vi "UHR-Fleezers Control (host) - 12.0.vi"() -> ()   [LabVIEW 2014] (continued)
            # "N total cycles"
            # "N steps"
            # "V_int"
            n2516 = local read "Scan Range (nm)"() -> (w4828:dbl)
            n2517 = local read "Number of F/B Scans (AOD)"() -> (w4845:u16)
            n2518 = Sign(1:w4828) -> (0:w4827:dbl)
            n2519 = Compound Arithmetic op=MULTIPLY(w4828, "MCL Step Position Ratio", "MCL/AOM Scale Tweak") -> (w4832:dbl)
            n2520 = Negate(x=w4827) -> (-x=w4824:dbl)
            n2521 = Multiply(x=w4824, y="MCL Step Increment (V_int)") -> (x*y=w4826:dbl)
            n2522 = Divide(x=w4832, y="MCL X Cal (nm/V)") -> (x/y=w4838:dbl)
            n2523 = Multiply(x=32767.0 ("y"), y=w4838) -> (x*y=w4844:dbl)
            n2524 = local read "Total Counts (ticks)"() -> (w4829:u32)
            n2525 = local read "Cycles/step (AOD)"() -> (w4840:u64)
            n2526 = local read "Scan steps (AOD)"() -> (w4841:u64)
            n2527 = Divide(x=w4844, y=10.0) -> (x/y=w4837:dbl)
            n2528 = Divide(x=w4837, y="MCL Step Increment (V_int)") -> (x/y=w4835:dbl)
            n2529 = Absolute Value(x=w4835) -> (abs(x)=w4823:dbl)
            n2530 = Compound Arithmetic op=MULTIPLY(w4841, w4840, w4829) -> (w4836:u64)
            n2531 = local write "wait to reset values"(w4851) -> ()
            n2532 = local write "MCL Scanning"(w4851) -> ()
            n2533 = Divide(x=w4836, y=w4823) -> (x/y=w4833:dbl)
            "MCL Count" <- w4833
            n2534 = xnode "Read/Write Control"("FPGA VI Reference In"=w4850, "error in"=w4849, "Scan steps (MCL)"=w4823, "Number of scans (MCL)"=w4845, "Cycles per step (MCL)"=u64 1, "Scan freq.  increment (MCL)"=w4826, "1D or 2D Scan?"=w4846, "MCL Scan Axis"=w4846, "Cont. Scan (MCL)"=w4846, "MCL count"=w4833) -> ("FPGA VI Reference Out"=w4848:T22, "error out"=w4847:errorcluster)
            n2535 = xnode "Read/Write Control"("FPGA VI Reference In"=w4848, "error in"=w4847, "AI to FIFO"=w4851, "APD to FIFO"=w4851, "Start scan"=w4851, "Start scan (MCL)"=w4851) -> ("FPGA VI Reference Out"=w4853:T22, "error out"=w4852:errorcluster)
          }
        }
        "Raster Scanning..." <- TRUE ("Scanning...")
      }
    }
    n2536 = local read "Flushing P3"() -> (w3628:bool)
    n2537 = case "Keep track of when Harvard Pump 3 is done flushing" shown="True" w3628 {
      frame False {
      }
      frame True {
        n2538 = local read "Flush rate (uL/m) P3"() -> (w4011:dbl)
        n2539 = local read "DMA Update Period (s)"() -> (w4005:dbl)
        n2540 = local read "HP3 Flush Time (s)"() -> (w4019:dbl)
        n2541 = Divide(x=w4011, y=60.0) -> (x/y=w4006:dbl)
        n2542 = feedback #6(0) -> (w4017:i32)
        n2543 = Increment(x=w4017) -> (x+1=w4012:i32)
        n2544 = Divide(x=w4019, y=w4005) -> (x/y=w4013:dbl)
        n2545 = Multiply(x=w4005, y=w4006) -> (x*y=w4004:dbl)
        n2546 = Greater?(x=w4012, y=w4013) -> (0:w4016:bool)
        n2547 = feedback #7(0.0) -> (w4007:dbl)
        n2548 = Compound Arithmetic op=MULTIPLY(w4005, w4012, w4006) -> (→"P3 Flush Volume (uL)":dbl)
        n2549 = case shown="True" w4016 {
          tunnel: w4012 -> [w4020 _]
          tunnel: [w4020 0] -> w4015
          frame False {
          }
          frame True {
            w4021 = FALSE ("Flushing P3")
            n2550 = local write "Inject Pump 3"(w4021) -> ()
            n2551 = local write "Flushing P3"(w4021) -> ()
            n2552 = property on="Clear Volume P3" class="Bool (strict)"("Val(Sgnl)"=TRUE ("Value (Signaling)")) -> ()  [unwired: 2 in, 2 out]
          }
        }
        n2553 = feedback-in #6(w4015) -> ()
        n2554 = Divide(x=w4012, y=w4013) -> (x/y=→"P3 Flushing Bar":dbl)
        n2555 = Add(x=w4004, y=w4007) -> (x+y=w4008:dbl)
        "Total Volume\nFlowed P3 (uL)" <- w4008
        n2556 = feedback-in #7(w4008) -> ()
      }
    }
    n2557 = And(x="Save scans", y=w3846) -> (x .and. y?=w3885:bool)
    n2558 = local read "Flushing samp"() -> (w3621:bool)
    n2559 = case shown="True" w3621 {
      frame False {
      }
      frame True {
        n2560 = local read "DMA Update Period (s)"() -> (w3964:dbl)
        n2561 = local read "Flush rate (mL/m)"() -> (w3976:dbl)
        n2562 = local read "Samp Flush Time (s)"() -> (w3977:dbl)
        n2563 = Divide(x=w3976, y=60.0) -> (x/y=w3963:dbl)
        n2564 = feedback #8(0) -> (w3969:i32)
        n2565 = Increment(x=w3969) -> (x+1=w3968:i32)
        n2566 = Divide(x=w3977, y=w3964) -> (x/y=w3973:dbl)
        n2567 = Multiply(x=w3964, y=w3963) -> (x*y=w3962:dbl)
        n2568 = Greater?(x=w3968, y=w3973) -> (0:w3972:bool)
        n2569 = feedback #9(0.0) -> (w3965:dbl)
        n2570 = Compound Arithmetic op=MULTIPLY(w3964, w3968, w3963) -> (→"Samp Volume (uL)":dbl)
        n2571 = Divide(x=w3968, y=w3973) -> (x/y=→"Samp flush bar":dbl)
        n2572 = case shown="True" w3972 {
          tunnel: [w3978 0] -> w3971
          tunnel: w3968 -> [w3978 _]
          frame False {
          }
          frame True {
            w3981 = FALSE ("Flushing samp")
            n2573 = local write "Sample Channel\nFlow"(w3981) -> ()
            n2574 = local write "Flushing samp"(w3981) -> ()
            n2575 = property on="Clear Volume" class="Bool (strict)"("Val(Sgnl)"=TRUE) -> ()  [unwired: 2 in, 2 out]
          }
        }
        n2576 = feedback-in #8(w3971) -> ()
        n2577 = Add(x=w3962, y=w3965) -> (x+y=w3966:dbl)
        "Total Volume\nFlowed Samp (uL)" <- w3966
        n2578 = feedback-in #9(w3966) -> ()
      }
    }
    n2579 = Compound Arithmetic op=OR("Start MCL Scan", "Confocal\nImage", "Confocal\nLinescan") -> (w3844:bool)
    n2580 = And(x="Save Data (MCL)", y=w3844) -> (x .and. y?=w3884:bool)
    n2581 = case "Start MCL raster scan" shown="True" w3844 {
      tunnel: w3612 -> [w4426 w4442]
      tunnel: w3886 -> [w4425 w4441]
      tunnel: [w4426 w4437] -> w3619
      tunnel: [w4425 w4436] -> w3617
      tunnel: [FALSE w4435] -> w3870
      tunnel: "Start MCL Scan" -> [_ w4430]
      tunnel: "Confocal\nImage" -> [_ w4429]
      tunnel: "Confocal\nLinescan" -> [_ _]
      frame False {
      }
      frame True {
        w4435 = TRUE
        n2582 = case shown="True" "Restart DMA? (MCL)" {
          tunnel: [w4487 w4489] -> w4440
          tunnel: [w4486 w4488] -> w4439
          tunnel: w4442 -> [w4487 w4492]
          tunnel: w4441 -> [w4486 w4491]
          frame False {
          }
          frame True {
            n2583 = call "reset FPGA DMA.vi"("error in"=w4491, "FPGA VI Reference In"=w4492) -> ("error out"=w4488:errorcluster, "FPGA VI Reference Out"=w4489:T22)
            n2584 = local write "Overflow (data lost)"(FALSE ("Overflow (data lost)")) -> ()
          }
        }
        n2585 = case shown="False" w4430 {
          selector: w4430 -> [_ w4446]
          tunnel: w4429 -> [w4445 _]
          tunnel: [w4445 w4446] -> w4428
          frame False {
            n2586 = property on="2D or 1D Scan" class="Bool (strict)"("Val(Sgnl)"=w4445) -> ()  [unwired: 2 in, 2 out]
            n2587 = property on="Confocal\nImage" class="Bool (strict)"("Value"=FALSE ("Start Confocal Map")) -> ()  [unwired: 2 in, 2 out]
          }
          frame True {
          }
        }
        n2588 = local write "MCL Scanning"(w4435) -> ()
        n2589 = local read "AO1"() -> (w4432:dbl)
        n2590 = local read "AO2"() -> (w4431:dbl)
        n2591 = case shown="True" "Center Scan" {
          tunnel: w4440 -> [w4453 w4485]
          tunnel: w4439 -> [w4452 w4484]
          tunnel: [w4451 w4483] -> w4437
          tunnel: [w4450 w4482] -> w4436
          tunnel: [w4448 w4469] -> w4434
          tunnel: [w4447 w4468] -> w4433
          tunnel: w4432 -> [w4448 w4474]
          tunnel: w4431 -> [w4447 w4477]
          tunnel: w4428 -> [_ _]
          frame False {
            w4449 = TRUE ("AI to FIFO")
            n2592 = xnode "Read/Write Control"("FPGA VI Reference In"=w4453, "error in"=w4452, "AI to FIFO"=w4449, "APD to FIFO"=w4449, "Start scan (MCL)"=w4449) -> ("FPGA VI Reference Out"=w4451:T22, "error out"=w4450:errorcluster)
          }
          frame True {
            w4481 = TRUE ("AI to FIFO")
            n2593 = local read "Scan steps (MCL)"() -> (w4460:u64)
            n2594 = local read "Scan lines (y)"() -> (w4456:u64)
            n2595 = local read "Fast Scan Dir"() -> (w4467:bool)
            n2596 = local read "Actual MCL Inc (V)"() -> (w4457:dbl)
            n2597 = Decrement(x=w4456) -> (x-1=w4455:u64)
            n2598 = Decrement(x=w4460) -> (x-1=w4459:u64)
            n2599 = Multiply(x=w4457, y=w4455) -> (x*y=w4454:dbl)
            n2600 = Divide(x=w4454, y=2.0) -> (x/y=w4464:dbl)
            n2601 = Multiply(x=w4457, y=w4459) -> (x*y=w4458:dbl)
            n2602 = Divide(x=w4458, y=2.0) -> (x/y=w4463:dbl)
            n2603 = Select(t=w4463, s=w4467, f=w4464) -> (s? t:f=w4462:dbl)
            n2604 = Select(t=w4464, s=w4467, f=w4463) -> (s? t:f=w4466:dbl)
            n2605 = Subtract(x=w4474, y=w4466) -> (x-y=w4465:dbl)
            n2606 = Subtract(x=w4477, y=w4462) -> (x-y=w4461:dbl)
            n2607 = local read "2D or 1D Scan"() -> (w4479:bool)
            n2608 = Not(x=w4467) -> (.not. x?=w4473:bool)
            n2609 = Not(x=w4479) -> (.not. x?=w4475:bool)
            n2610 = And(x=w4467, y=w4475) -> (x .and. y?=w4476:bool)
            n2611 = And(x=w4475, y=w4473) -> (x .and. y?=w4478:bool)
            n2612 = Select(t=w4477, s=w4478, f=w4461) -> (s? t:f=w4468:dbl)
            n2613 = Select(t=w4474, s=w4476, f=w4465) -> (s? t:f=w4469:dbl)
            n2614 = call "Volt to I16.vi"("Voltage In"=w4469) -> ("I16 Voltage Out"=w4472:i16)
            n2615 = call "Volt to I16.vi"("Voltage In"=w4468) -> ("I16 Voltage Out"=w4471:i16)
            n2616 = xnode "Read/Write Control"("FPGA VI Reference In"=w4485, "error in"=w4484, "AI to FIFO"=w4481, "APD to FIFO"=w4481, "Start scan (MCL)"=w4481, "AO1"=w4472, "AO2"=w4471) -> ("FPGA VI Reference Out"=w4483:T22, "error out"=w4482:errorcluster)
          }
        }
        "Initial Y" <- w4434
        "Initial X" <- w4433
        n2617 = local write "Tab Control 6"(T3."Imaging" ("Tab Control 6")) -> ()
        "wait to reset values" <- w4435
      }
    }
    n2618 = case shown="True" "Wiggle" {
      selector: "Wiggle" -> [w3935 _]
      tunnel: w3619 -> [w3937 w3950]
      tunnel: [w3934 w3953] -> w3618
      tunnel: w3617 -> [w3936 w3948]
      tunnel: [w3933 w3952] -> w3616
      frame False {
        n2619 = xnode "Read/Write Control"("FPGA VI Reference In"=w3937, "error in"=w3936, "Wiggle trap 1"=w3935) -> ("FPGA VI Reference Out"=w3934:T22, "error out"=w3933:errorcluster)
      }
      frame True {
        w3942 = FALSE ("Abort wiggle")
        w3946 = TRUE
        n2620 = local read "Restart DMA? (AOD)"() -> (w3951:bool)
        n2621 = case shown="True" w3951 {
          tunnel: w3950 -> [w3955 w3960]
          tunnel: [w3955 w3959] -> w3949
          tunnel: w3948 -> [w3954 w3958]
          tunnel: [w3954 w3957] -> w3947
          frame False {
          }
          frame True {
            n2622 = local write "Overflow (data lost)"(FALSE) -> ()
            n2623 = call "reset FPGA DMA.vi"("error in"=w3958, "FPGA VI Reference In"=w3960) -> ("error out"=w3957:errorcluster, "FPGA VI Reference Out"=w3959:T22)
          }
        }
        n2624 = local write "Wiggle"(FALSE) -> ()
        n2625 = xnode "Read/Write Control"("FPGA VI Reference In"=w3949, "error in"=w3947, "AI to FIFO"=w3946, "APD to FIFO"=w3946, "Wiggle trap 1"="Wiggle T1", "Wiggle freq 1 (Hz)"="Wiggle freq 1 (Hz)", "Wiggle amp 1"="Wiggle amp 1 (units?)", "Abort wiggle 1"=w3942, "Wiggle trap 2"="Wiggle T2", "Abort wiggle 2"=w3942, "Wiggle freq 2 (Hz)"="Wig Freq 2 (Hz)", "Wiggle amp 2"="Wig amp 2") -> ("FPGA VI Reference Out"=w3953:T22, "error out"=w3952:errorcluster)
      }
    }
    n2626 = local read "Trap Pos Elements/DMA read"() -> (w3602:u32)
    n2627 = local read "Trap AI Elements/DMA read"() -> (w3596:u32)
    n2628 = local read "APD Elements/DMA read"() -> (w3604:u32)
    n2629 = xnode "Get APD Data"("FPGA VI Reference In"=w3618, "error in"=w3616, "Number of Elements"=w3604, "Timeout (ms)"=-1) -> ("Data"=w3780:u32[], "Elements Remaining"=→"APD FIFO Elements Remaining":u32)  [unwired: 2 out]
    n2630 = xnode "Invoke Method"("FPGA VI Reference In"=w3618, "error in"=w3616, "Number of Elements"=w3602, "Timeout (ms)"=-1) -> ("Data"=w3711:u16[], "Elements Remaining"=→"Trap Pos FIFO El Remaining":u32)  [unwired: 2 out]
    n2631 = xnode "Get Trap Data"("FPGA VI Reference In"=w3618, "error in"=w3616, "Number of Elements"=w3596, "Timeout (ms)"=-1 ("Timeout")) -> ("FPGA VI Reference Out"=w3649:T22, "error out"=w3648:errorcluster, "Data"=w3712:i16[], "Elements Remaining"=w3595:u32)
    "FIFO El. Rem." <- w3595
    n2632 = local read "Trap AI FIFO Depth"() -> (w3930:u32)
    n2633 = Subtract(x=w3930, y=w3596) -> (x-y=w3929:u32)
    n2634 = Decimate 1D Array(w3711) -> (w3600:u16[], w3598:u16[], w3599:u16[])
    n2635 = Divide(x=w3595, y=w3929) -> (x/y=w3928:dbl)
    "Buffer Status" <- w3928
    n2636 = To Unsigned Long Integer(number=w3600) -> (unsigned 32bit integer=w3710:u32[])
    n2637 = Join Numbers(hi=w3598, lo=w3599) -> ((hi.lo)=w3709:u32[])
    n2638 = Equal?(x=w3928, y=1.0) -> (x = y?=w3926:bool)
    n2639 = Join Numbers(hi=w3710, lo=w3709) -> ((hi.lo)=w3703:u64[])
    n2640 = call "IR AOM word to freq - vec.vi"("Frequency Word In (double vec)"=w3703) -> ("Frequency Out"=w3746:dbl[])
    n2641 = case "Alert buffer overflow" shown="True" w3926 {
      frame False {
      }
      frame True {
        n2642 = call <vilib>:"Beep.vi"() -> ()  [unwired: 3 in, 9 out]
        "Overflow (data lost)" <- TRUE ("Overflow (data lost)")
      }
    }
    n2643 = Decimate 1D Array(w3746) -> (w3745:dbl[], w3744:dbl[])
    n2644 = Build Array(w3745, w3744) -> (w3743:dbl[][])
    n2645 = local read "Trap Sets"() -> (w3810:u32)
    n2646 = case "Deinterlace trap data, average down PSD" shown="2" w3810 {
      tunnel: w3712 -> [w4518 w4587]
      tunnel: [w4521 w4584] -> w3803
      tunnel: [w4518 w4586] -> w3706
      tunnel: "Detector Type" -> [w4523 w4582]
      tunnel: [w4522 w4585] -> w3802
      tunnel: [w4520 w4583] -> w3903
      frame 1, Default {
        n2647 = Divide(x=w4518, y=3276.7) -> (x/y=w4519:dbl[])
        n2648 = Decimate 1D Array(w4519) -> (w4532:dbl[], w4531:dbl[], w4530:dbl[], w4529:dbl[], w4528:dbl[], w4527:dbl[], w4526:dbl[], w4525:dbl[])
        n2649 = case shown="\"IR-QPD + PSD + FB-QPD position\"" w4523 {
          tunnel: w4532 -> [w4556 w4581]
          tunnel: w4531 -> [w4555 w4580]
          tunnel: w4530 -> [w4540 w4558]
          tunnel: w4529 -> [w4541 w4568]
          tunnel: w4528 -> [w4554 w4579]
          tunnel: w4527 -> [w4553 w4578]
          tunnel: w4526 -> [w4537 w4559]
          tunnel: w4525 -> [w4536 w4557]
          tunnel: [w4535 w4565] -> w4522
          tunnel: [w4534 w4564] -> w4521
          tunnel: [w4533 w4563] -> w4520
          frame "IR-QPD + PSD + FB-QPD", Default {
            w4533 = 0  # Channel pattern
            n2650 = Divide(x=w4556, y=w4541) -> (x/y=w4543:dbl[])
            n2651 = Divide(x=w4555, y=w4541) -> (x/y=w4542:dbl[])
            n2652 = Divide(x=w4554, y=w4537) -> (x/y=w4539:dbl[])
            n2653 = Divide(x=w4553, y=w4536) -> (x/y=w4538:dbl[])
            n2654 = Build Array(w4543, w4542, w4541, w4540, w4539, w4538, w4537, w4536) -> (w4534:dbl[][])
            n2655 = Bundle("T1 Y", "T1 X", "T1 Sum", "FB Sum", "PSD Y", "PSD X", "PSD Y Sum", "PSD X Sum") -> (w4552:T47)  [unwired: 1 out]
            n2656 = Cluster To Array(cluster=w4552) -> (array=w4535:string[])
          }
          frame "IR-QPD + PSD + FB-QPD position" {
            w4563 = 3  # Channel pattern
            n2657 = Negate(x=w4559) -> (-x=w4560:dbl[])
            n2658 = Divide(x=w4581, y=w4568) -> (x/y=w4570:dbl[])
            n2659 = Divide(x=w4580, y=w4568) -> (x/y=w4569:dbl[])
            n2660 = Divide(x=w4579, y=w4559) -> (x/y=w4567:dbl[])
            n2661 = Divide(x=w4578, y=w4560) -> (x/y=w4566:dbl[])
            n2662 = Build Array(w4570, w4569, w4568, w4557, w4558, w4567, w4566, w4559) -> (w4564:dbl[][])
            n2663 = Bundle("T1 Y", "T1 X", "T1 Sum", "FB X", "FB Sum", "PSD Y", "PSD X", "PSD Y Sum") -> (w4577:T47)  [unwired: 1 out]
            n2664 = Cluster To Array(cluster=w4577) -> (array=w4565:string[])
          }
        }
      }
      frame 2 {
        n2665 = case shown="\"IR-QPD + PSD + FB-QPD XY positions\"" w4582 {
          tunnel: w4587 -> [w4649 w4716 w4785]
          tunnel: [w4600 w4712 w4730] -> w4586
          tunnel: [w4625 w4704 w4771] -> w4585
          tunnel: [w4624 w4671 w4742] -> w4584
          tunnel: [w4620 w4702 w4769] -> w4583
          frame "IR-QPD + PSD + FB-QPD", Default {
            w4620 = 1  # Channel pattern
            # "time average x2 the 4th signal and the 4 psd signals (detection laser)"
            # "deinterlace 3 signals from qpd"
            n2666 = Decimate 1D Array(w4649) -> (w4648:i16[], w4647:i16[], w4623:i16[], w4646:i16[], w4599:i16[], w4598:i16[], w4597:i16[], w4596:i16[])
            n2667 = Decimate 1D Array(w4623) -> (w4589:i16[], w4588:i16[])
            n2668 = Decimate 1D Array(w4648) -> (w4595:i16[], w4594:i16[])
            n2669 = Decimate 1D Array(w4647) -> (w4593:i16[], w4591:i16[])
            n2670 = Decimate 1D Array(w4646) -> (w4592:i16[], w4590:i16[])
            n2671 = call "downsample 1D array - double.vi"("Ave N"=2.0, "Array In"=w4599) -> ("Array Out"=w4641:dbl[])  [unwired: 1 out]
            n2672 = call "downsample 1D array - double.vi"("Ave N"=2.0, "Array In"=w4598) -> ("Array Out"=w4626:dbl[])  [unwired: 1 out]
            n2673 = call "downsample 1D array - double.vi"("Ave N"=2.0, "Array In"=w4597) -> ("Array Out"=w4640:dbl[])  [unwired: 1 out]
            n2674 = call "downsample 1D array - double.vi"("Ave N"=2.0, "Array In"=w4596) -> ("Array Out"=w4639:dbl[])  [unwired: 1 out]
            n2675 = Interleave 1D Arrays(w4595, w4593, w4592, w4594, w4591, w4590, w4589, w4588, w4641, w4626, w4640, w4639) -> (w4638:dbl[])
            n2676 = Divide(x=w4638, y=3276.7) -> (x/y=w4637:dbl[])
            n2677 = Decimate 1D Array(w4637) -> (w4636:dbl[], w4635:dbl[], w4634:dbl[], w4633:dbl[], w4632:dbl[], w4631:dbl[], w4622:dbl[], w4621:dbl[], w4630:dbl[], w4629:dbl[], w4628:dbl[], w4627:dbl[])
            n2678 = Divide(x=w4636, y=w4634) -> (x/y=w4607:dbl[])
            n2679 = Divide(x=w4635, y=w4634) -> (x/y=w4606:dbl[])
            n2680 = Divide(x=w4633, y=w4631) -> (x/y=w4605:dbl[])
            n2681 = Divide(x=w4632, y=w4631) -> (x/y=w4604:dbl[])
            n2682 = Divide(x=w4630, y=w4628) -> (x/y=w4603:dbl[])
            n2683 = Divide(x=w4629, y=w4627) -> (x/y=w4602:dbl[])
            n2684 = Build Array(w4607, w4606, w4634, w4605, w4604, w4631, w4622, w4621, w4603, w4602, w4628, w4627) -> (w4624:dbl[][])
            n2685 = Bundle("T1 Y", "T1 X", "T1 Sum", "T2 Y", "T2 X", "T2 Sum", "T1 FB Sum", "T2 FB Sum", "PSD Y", "PSD X", "PSD Y Sum", "PSD X Sum") -> (w4608:T48)  [unwired: 1 out]
            n2686 = To Word Integer(number=w4638) -> (16bit integer=w4600:i16[])
            n2687 = Cluster To Array(cluster=w4608) -> (array=w4625:string[])
          }
          frame "IR-QPD + PSD + FB-QPD X position" {
            w4702 = 2  # Channel pattern
            # "time average x2 the 3 psd signals (detection laser)"
            # "deinterlace 3 signals from qpds"
            n2688 = Decimate 1D Array(w4716) -> (w4715:i16[], w4714:i16[], w4703:i16[], w4713:i16[], w4663:i16[], w4662:i16[], w4661:i16[], w4690:i16[])
            n2689 = Decimate 1D Array(w4703) -> (w4653:i16[], w4651:i16[])
            n2690 = Decimate 1D Array(w4715) -> (w4660:i16[], w4657:i16[])
            n2691 = Decimate 1D Array(w4714) -> (w4659:i16[], w4656:i16[])
            n2692 = Decimate 1D Array(w4713) -> (w4658:i16[], w4655:i16[])
            n2693 = Decimate 1D Array(w4690) -> (w4654:i16[], w4652:i16[])
            n2694 = call "downsample 1D array - I16.vi"("Ave N"=2.0, "Array In"=w4663) -> ("Array Out"=w4668:i16[])  [unwired: 1 in]
            n2695 = call "downsample 1D array - I16.vi"("Ave N"=2.0, "Array In"=w4661) -> ("Array Out"=w4664:i16[])  [unwired: 1 in]
            n2696 = call "downsample 1D array - I16.vi"("Ave N"=2.0, "Array In"=w4662) -> ("Array Out"=w4666:i16[])  [unwired: 1 in]
            n2697 = Interleave 1D Arrays(w4660, w4659, w4658, w4657, w4656, w4655, w4654, w4653, w4652, w4651, w4668, w4666, w4664) -> (w4712:i16[])
            n2698 = Divide(x=w4712, y=3276.7) -> (x/y=w4711:dbl[])
            n2699 = Decimate 1D Array(w4711) -> (w4710:dbl[], w4709:dbl[], w4708:dbl[], w4707:dbl[], w4706:dbl[], w4705:dbl[], w4682:dbl[], w4680:dbl[], w4679:dbl[], w4677:dbl[], w4676:dbl[], w4675:dbl[], w4672:dbl[])
            n2700 = Negate(x=w4672) -> (-x=w4670:dbl[])
            n2701 = Divide(x=w4676, y=w4672) -> (x/y=w4674:dbl[])
            n2702 = Divide(x=w4675, y=w4670) -> (x/y=w4673:dbl[])
            n2703 = Divide(x=w4710, y=w4708) -> (x/y=w4694:dbl[])
            n2704 = Divide(x=w4709, y=w4708) -> (x/y=w4693:dbl[])
            n2705 = Divide(x=w4707, y=w4705) -> (x/y=w4692:dbl[])
            n2706 = Divide(x=w4706, y=w4705) -> (x/y=w4691:dbl[])
            n2707 = Divide(x=w4682, y=w4680) -> (x/y=w4681:dbl[])
            n2708 = Divide(x=w4679, y=w4677) -> (x/y=w4678:dbl[])
            n2709 = Build Array(w4694, w4693, w4708, w4692, w4691, w4705, w4681, w4680, w4678, w4677, w4674, w4673, w4672) -> (w4671:dbl[][])
            n2710 = Bundle("T1 Y", "T1 X", "T1 Sum", "T2 Y", "T2 X", "T2 Sum", "T1 FB X", "T1 FB Sum", "T2 FB X", "T2 FB Sum", "PSD Y", "PSD X", "PSD Y Sum") -> (w4695:T49)  [unwired: 1 out]
            n2711 = Cluster To Array(cluster=w4695) -> (array=w4704:string[])
          }
          frame "IR-QPD + PSD + FB-QPD XY positions" {
            w4769 = 4  # Channel pattern
            # "time average x2 the 3 psd signals (detection laser)"
            # "deinterlace 3 signals from qpds"
            n2712 = Decimate 1D Array(w4785) -> (w4784:i16[], w4783:i16[], w4770:i16[], w4782:i16[], w4740:i16[], w4758:i16[])  [unwired: 2 out]
            n2713 = Decimate 1D Array "Feedback Sum"(w4770) -> (w4721:i16[], w4718:i16[])
            n2714 = Decimate 1D Array "QPD Y"(w4784) -> (w4729:i16[], w4726:i16[])
            n2715 = Decimate 1D Array "QPD X"(w4783) -> (w4728:i16[], w4725:i16[])
            n2716 = Decimate 1D Array "Feedback Y"(w4740) -> (w4723:i16[], w4720:i16[])
            n2717 = Decimate 1D Array "QPD Sum"(w4782) -> (w4727:i16[], w4724:i16[])
            n2718 = Decimate 1D Array "Feedback X"(w4758) -> (w4722:i16[], w4719:i16[])
            n2719 = call "downsample 1D array - double.vi"("Ave N"=2.0) -> ("Array Out"=w4757:dbl[])  [unwired: 1 in, 1 out]
            n2720 = call "downsample 1D array - double.vi"("Ave N"=2.0) -> ("Array Out"=w4756:dbl[])  [unwired: 1 in, 1 out]
            n2721 = Interleave 1D Arrays(w4729, w4728, w4727, w4726, w4725, w4724, w4723, w4722, w4721, w4720, w4719, w4718, w4757, w4756) -> (w4779:dbl[])
            n2722 = Divide(x=w4779, y=3276.7) -> (x/y=w4778:dbl[])
            n2723 = Decimate 1D Array(w4778) -> (w4777:dbl[], w4776:dbl[], w4775:dbl[], w4774:dbl[], w4773:dbl[], w4772:dbl[], w4737:dbl[], w4749:dbl[], w4735:dbl[], w4736:dbl[], w4747:dbl[], w4733:dbl[], w4745:dbl[], w4743:dbl[])
            n2724 = Negate(x=w4743) -> (-x=w4741:dbl[])
            n2725 = Divide(x=w4745, y=w4741) -> (x/y=w4744:dbl[])
            n2726 = Divide(x=w4736, y=w4733) -> (x/y=w4732:dbl[])
            n2727 = Divide(x=w4737, y=w4735) -> (x/y=w4734:dbl[])
            n2728 = Divide(x=w4777, y=w4775) -> (x/y=w4762:dbl[])
            n2729 = Divide(x=w4776, y=w4775) -> (x/y=w4761:dbl[])
            n2730 = Divide(x=w4774, y=w4772) -> (x/y=w4760:dbl[])
            n2731 = Divide(x=w4773, y=w4772) -> (x/y=w4759:dbl[])
            n2732 = Divide(x=w4749, y=w4735) -> (x/y=w4748:dbl[])
            n2733 = Divide(x=w4747, y=w4733) -> (x/y=w4746:dbl[])
            n2734 = Build Array(w4762, w4761, w4775, w4760, w4759, w4772, w4734, w4748, w4735, w4732, w4746, w4733, w4744, w4743) -> (w4742:dbl[][])
            n2735 = Bundle("T1 Y", "T1 X", "T1 Sum", "T2 Y", "T2 X", "T2 Sum", "T1 FB Y", "T1 FB X", "T1 FB Sum", "T2 FB Y", "T2 FB X", "T2 FB Sum", "PSD X", "PSD Y Sum") -> (w4731:T50)  [unwired: 1 out]
            n2736 = To Word Integer(number=w4779) -> (16bit integer=w4730:i16[])
            n2737 = Cluster To Array(cluster=w4731) -> (array=w4771:string[])
          }
        }
      }
    }
    "AI labels" <- w3802
    n2738 = Decimate 1D Array(w3780) -> (w3590:u32[], w3591:u32[])
    n2739 = local read "DMA Update Period (s)"() -> (w3811:dbl)
    n2740 = Build Array(w3590, w3591) -> (w3594:u32[][])
    n2741 = local read "Data Period (s)"() -> (w3665:dbl)
    n2742 = local read "BD 1 Frequency 2 (MHz)"() -> (w3698:dbl)
    n2743 = local read "BD 1 Frequency 1 (MHz)"() -> (w3699:dbl)
    n2744 = Decimate 1D Array(w3706) -> (w3726:i16[], w3725:i16[], w3723:i16[], w3722:i16[])  [unwired: 9 out]
    n2745 = To Double Precision Float(number=w3594) -> (double precision float=w3868:dbl[][])
    n2746 = local read "APD Integration Time (s)"() -> (w3762:dbl)
    n2747 = Multiply(x=w3665, y="Trap Pos. Disp. Downsample") -> (x*y=w3663:dbl)
    n2748 = Divide(x=w3726, y=w3725) -> (x/y=w3727:dbl[])
    n2749 = Divide(x=w3723, y=w3722) -> (x/y=w3724:dbl[])
    n2750 = feedback #10(0.0) -> (w3740:dbl)
    n2751 = Add(x=w3811, y=w3740) -> (x+y=w3905:dbl)
    n2752 = feedback-in #10(w3905) -> ()
    n2753 = local read "AOM X Cal (nm/MHz)"() -> (w3696:dbl)
    n2754 = To Time Stamp(1:w3740) -> (0:w3739:timestamp)
    n2755 = Split 1D Array(array=w3727, index="N El. to Ave.") -> (second subarray=w3730:dbl[])  [unwired: 1 out]
    n2756 = Split 1D Array(array=w3724, index="N El. to Ave.") -> (second subarray=w3729:dbl[])  [unwired: 1 out]
    n2757 = Multiply(x=w3665, y="Trap Disp. Downsample") -> (x*y=w3741:dbl)
    "Display Period (s)" <- w3741
    n2758 = for "Trap AI" {
      tunnel: [w4517] -> w3899 mode=indexing
      tunnel: w3739 -> [w4507]
      tunnel: "Trap Disp. Downsample" -> [w4515]
      tunnel: w3803 -> [w4513] mode=indexing
      tunnel: w3665 -> [w4512]
      tunnel: w3802 -> [w4511] mode=indexing
      tunnel: w3738 -> [w4510]
      tunnel: [w4509] -> w3772 mode=indexing
      tunnel: w3741 -> [w4508]
      workers-P: _ -> [_]
      n2759 = Bundle By Name("Y"=w4513, "dt"=w4512) -> (w4514:waveform(dbl))  [unwired: 1 out]
      n2760 = Set Waveform Attribute(5:w4511, 6:w4510, 7:w4514) -> (3:w4509:waveform(dbl))  [unwired: 1 in, 2 out]
      n2761 = call "downsample 1D array - double.vi"("Ave N"=w4515, "Array In"=w4513) -> ("Array Out"=w4516:dbl[])  [unwired: 1 out]
      n2762 = Bundle By Name(cluster=w4509, "t0"=w4507, "Y"=w4516, "dt"=w4508) -> (w4517:waveform(dbl))
    }
    n2763 = Bundle("BD 1 Frequency 1 (MHz)"=w3699, "BD 1 Frequency 2 (MHz)"=w3698) -> (w3700:T51)  [unwired: 1 out]
    n2764 = call-poly <vilib>:"Mean.vi"("X"=w3729) -> ("mean"=w3717:dbl)  [unwired: 1 out]
    n2765 = call-poly <vilib>:"Mean.vi"("X"=w3730) -> ("mean"=w3718:dbl)  [unwired: 1 out]
    n2766 = Reciprocal(x=w3741) -> (1/x=→"Trap Disp. Freq. (Hz)":dbl)
    n2767 = Cluster To Array(cluster=w3700) -> (array=w3697:dbl[])
    n2768 = local read "Trap X AI1 (DMA)"() -> (w3728:T13)
    n2769 = local read "Data points/scans (MCL)"() -> (w3879:dbl)
    n2770 = To Fixed-Point(number=w3717) -> (fixed-point=w3715:fxp<+/-,16,1>)  [unwired: 1 in]
    n2771 = To Fixed-Point(number=w3718) -> (fixed-point=w3716:fxp<+/-,16,1>)  [unwired: 1 in]
    n2772 = Bundle("Trap 1 Pos.", "Trap 2 Pos.") -> (w3737:cluster{string, string})  [unwired: 1 out]
    n2773 = Bundle By Name(cluster=w3728, "Set 1"=w3716, "Set 2"=w3715) -> (→"Trap X AI1 (DMA)":T13)
    n2774 = Cluster To Array(cluster=w3737) -> (array=w3734:string[])
    n2775 = Bundle("APD 1", "APD 2") -> (w3898:cluster{string, string})  [unwired: 1 out]
    n2776 = Select(t=-1.0, s="Negate Y Axis", f=1.0) -> (s? t:f=w3682:dbl)
    n2777 = for "Trap Position" {
      tunnel: w3743 -> [w4149] mode=indexing
      tunnel: "Trap Pos. Disp. Downsample" -> [w4148]
      tunnel: w3663 -> [w4146]
      tunnel: w3739 -> [w4145]
      tunnel: w3738 -> [w4143]
      tunnel: w3734 -> [w4142] mode=indexing
      tunnel: [w4141] -> w3652 mode=indexing
      tunnel: w3697 -> [w4139] mode=indexing
      tunnel: w3696 -> [w4137]
      tunnel: w3682 -> [w4136]
      n2778 = call "downsample 1D array - double.vi"("Ave N"=w4148, "Array In"=w4149) -> ("Array Out"=w4147:dbl[])  [unwired: 1 out]
      n2779 = Subtract(x=w4147, y=w4139) -> (x-y=w4140:dbl[])
      n2780 = Multiply(x=w4137, y=w4140) -> (x*y=w4138:dbl[])
      n2781 = Multiply(x=w4136, y=w4138) -> (x*y=w4135:dbl[])
      n2782 = Bundle By Name("Y"=w4135, "dt"=w4146, "t0"=w4145) -> (w4144:waveform(dbl))  [unwired: 1 out]
      n2783 = Set Waveform Attribute(5:w4142, 6:w4143, 7:w4144) -> (3:w4141:waveform(dbl))  [unwired: 1 in, 2 out]
    }
    n2784 = Cluster To Array(cluster=w3898) -> (array=w3895:string[])
    n2785 = for "APD" {
      tunnel: w3868 -> [w4493] mode=indexing
      tunnel: w3762 -> [w4504]
      tunnel: [w4500] -> w3768 mode=indexing
      tunnel: "APD Disp. Scale" -> [w4501]
      tunnel: w3738 -> [w4499]
      tunnel: w3895 -> [w4498] mode=indexing
      tunnel: "APD Disp. Downsample" -> [w4495]
      tunnel: [w4497] -> w3894
      workers-P: _ -> [_]
      tunnel: w3739 -> [w4494]
      n2786 = call "integrate 1D array interval - double.vi"("Ave N"=w4495, "Array In"=w4493) -> ("Array Out"=w4496:dbl[])  [unwired: 1 out]
      n2787 = Multiply(x=w4504, y=w4495) -> (x*y=w4497:dbl)
      n2788 = Divide(x=w4496, y=w4501) -> (x/y=w4502:dbl[])
      n2789 = Bundle By Name("t0"=w4494, "Y"=w4502, "dt"=w4497) -> (w4503:waveform(dbl))  [unwired: 1 out]
      n2790 = Set Waveform Attribute(5:w4498, 6:w4499, 7:w4503) -> (3:w4500:waveform(dbl))  [unwired: 1 in, 2 out]
    }
    "APD Display Period (s)" <- w3894
    n2791 = Reciprocal(x=w3894) -> (1/x=→"APD Display Freq. (Hz)":dbl)
    n2792 = local read "Display Period (s)"() -> (w3789:dbl)
    n2793 = Increment(x=w3879) -> (x+1=w3880:dbl)
    n2794 = To Double Precision Float(number=w3590) -> (double precision float=w3800:dbl[])
    n2795 = Index Array(array=w3652, index=0) -> (element=w3656:waveform(dbl))
    n2796 = Index Array(array=w3652, index=1) -> (element=w3651:waveform(dbl))
    n2797 = feedback #11(w3880) -> (w3883:dbl)
    n2798 = Select(t=0, s=w3870, f=w3883) -> (s? t:f=w3876:dbl)
    n2799 = Array Size(array=w3800) -> (size(s)=w3882:i32)
    n2800 = Add(x=w3882, y=w3876) -> (x+y=w3877:dbl)
    n2801 = Unbundle By Name(w3656) -> ("Y"=w3657:dbl[])
    n2802 = feedback #12(w3590) -> (w3867:u32[])
    n2803 = Build Array (concatenate)(w3867, w3590) -> (w3864:u32[])
    n2804 = feedback #13(w3591) -> (w3767:u32[])
    n2805 = Divide(x="Bead Sep. Int. Time (s)", y=w3789) -> (x/y=w3692:dbl)
    n2806 = Build Array (concatenate)(w3767, w3591) -> (w3766:u32[])
    n2807 = Add(x=w3657, y="FB Trap Pos Offset") -> (x+y=w3655:dbl[])
    "T1 x pos data" <- w3655
    n2808 = Greater?(x=w3877, y=w3879) -> (0:w3878:bool)
    n2809 = feedback #14(w3655) -> (w3694:dbl[])
    n2810 = Build Array (concatenate)(w3655, w3694) -> (w3693:dbl[])
    n2811 = Bundle By Name(cluster=w3656, "Y"=w3655) -> (w3654:waveform(dbl))
    n2812 = Select(t=w3876, s=w3878, f=w3877) -> (s? t:f=w3875:dbl)
    n2813 = feedback-in #11(w3875) -> ()
    n2814 = Array Size(array=w3864) -> (size(s)=w3861:i32)
    n2815 = Array Size(array=w3590) -> (size(s)=w3863:i32)
    n2816 = local read "MCL Scanning"() -> (w3873:bool)
    n2817 = local read "APD Integration Time (s)"() -> (w3775:dbl)
    n2818 = Bundle(w3654, w3651) -> (w3650:cluster{waveform(dbl), waveform(dbl)})  [unwired: 1 out]
    n2819 = Build Array (concatenate)(w3768, w3899) -> (w3770:waveform(dbl)[])
    "All Signals" <- w3770
    n2820 = Split 1D Array(array=w3693, index=w3692) -> (first subarray=w3686:dbl[])  [unwired: 1 out]
    n2821 = feedback-in #14(w3686) -> ()
    n2822 = Multiply(x=w3863, y="APD Ave N") -> (x*y=w3862:dbl)
    n2823 = Greater?(x=w3861, y=w3862) -> (0:w3865:bool)
    n2824 = Not(x=w3878) -> (.not. x?=w3872:bool)
    n2825 = Cluster To Array(cluster=w3650) -> (array=w3626:waveform(dbl)[])
    "Trap Positions" <- w3626
    n2826 = To Double Precision Float(number=w3591) -> (double precision float=w3749:dbl[])
    n2827 = call-poly <vilib>:"Mean.vi"("X"=w3686) -> ("mean"=w3685:dbl)  [unwired: 1 out]
    "Mean T1 Position (nm)" <- w3685
    n2828 = Subtract(x=w3686, y=w3685) -> (x-y=w3691:dbl[])
    n2829 = Square(x=w3691) -> (x^2=w3690:dbl[])
    n2830 = And(x=w3872, y=w3873) -> (x .and. y?=w3874:bool)
    n2831 = call-poly <vilib>:"Mean.vi"("X"=w3690) -> ("mean"=w3689:dbl)  [unwired: 1 out]
    n2832 = case shown="True" w3865 {
      tunnel: w3864 -> [w4276 w4278]
      tunnel: [w4276 w4282] -> w3592
      tunnel: w3862 -> [_ w4280]
      tunnel: w3861 -> [_ w4283]
      tunnel: w3766 -> [w4275 w4277]
      tunnel: [w4275 w4279] -> w3593
      frame False {
      }
      frame True {
        n2833 = Subtract(x=w4283, y=w4280) -> (x-y=w4281:dbl)
        n2834 = Array Subset(array=w4278, index=w4281, length=w4280) -> (w4282:u32[])
        n2835 = Array Subset(array=w4277, index=w4281, length=w4280) -> (w4279:u32[])
      }
    }
    n2836 = feedback-in #12(w3592) -> ()
    n2837 = feedback-in #13(w3593) -> ()
    n2838 = Square Root(x=w3689) -> (sqrt(x)=w3688:dbl)
    n2839 = Or(x=w3874, y=w3870) -> (x .or. y?=w3871:bool)
    n2840 = Equal?(x="Tab Control 6", y=T41."High Res Display") -> (x = y?=w3806:bool)
    n2841 = Multiply(x="APD Disp. Scale", y=w3768) -> (x*y=w3777:waveform(dbl)[])
    n2842 = Multiply(x=10.0, y=w3688) -> (x*y=→"Trap 1 Position RMS (A)":dbl)
    n2843 = Multiply(x="APD Disp. Downsample", y=w3775) -> (x*y=w3773:dbl)
    n2844 = Divide(x=w3777, y=w3773) -> (x/y=w3747:waveform(dbl)[])
    n2845 = case "For displaying the high resolution display (no downsampling)" shown="True" w3806 {
      tunnel: w3772 -> [_ w4174]
      frame False {
      }
      frame True {
        n2846 = Index Array(array=w4174, index="High Res. Display") -> (element=w4175:waveform(dbl))
        n2847 = call <vilib>:"Std Deviation and Variance.vi"("X"=w4175) -> ("mean"=w4182:dbl, "standard deviation"=w4187:dbl)  [unwired: 1 in, 1 out]
        "Mean Intensity" <- w4182
        "Sigma" <- w4187
        n2848 = Subtract(x=w4175, y=w4182) -> (x-y=w4181:waveform(dbl))
        n2849 = Select(t=w4181, s="Subtract mean", f=w4175) -> (s? t:f=→"1 Channel":waveform(dbl))
        n2850 = Divide(x=w4187, y=w4182) -> (x/y=→"Sigma/Mean":dbl)
        n2851 = feedback #15(1) -> (w4176:i32)
        n2852 = Greater Or Equal?(x=w4176, y="Slow mean N ave.") -> (x >= y?=w4189:bool)
        n2853 = Increment(x=w4176) -> (x+1=w4191:i32)
        n2854 = Select(t=1, s=w4189, f=w4191) -> (s? t:f=w4178:i32)
        n2855 = feedback-in #15(w4178) -> ()
        n2856 = feedback #16() -> (w4179:waveform(dbl))  [unwired: 1 out]
        n2857 = case shown="Default" w4176 {
          tunnel: [w4194 w4197] -> w4180
          tunnel: w4179 -> [w4196 _]
          tunnel: w4175 -> [w4195 w4197]
          frame Default {
            n2858 = call-poly <vilib>:"Append Waveforms.vi"("waveform B"=w4195, "waveform A"=w4196) -> ("waveform out"=w4194:waveform(dbl))  [unwired: 1 in, 8 out]
          }
          frame 1 {
          }
        }
        n2859 = feedback-in #16(w4180) -> ()
        n2860 = case shown="True" w4189 {
          tunnel: w4180 -> [_ w4193]
          frame False {
          }
          frame True {
            n2861 = call-poly <vilib>:"Mean.vi"("X"=w4193) -> ("mean"=→"Slow mean":dbl)  [unwired: 1 out]
          }
        }
      }
    }
    n2862 = Index Array(array=w3747, index=0) -> (element=w3756:waveform(dbl))
    n2863 = Index Array(array=w3747, index=1) -> (element=w3754:waveform(dbl))
    n2864 = case "For computing FFTs for display" shown="True" "Compute FFT" {
      tunnel: w3772 -> [_ w4888]
      frame False {
      }
      frame True {
        n2865 = Build Array("FFT 1 Choice 1", "FFT 1 Choice 2", "FFT 2 Choice 1", "FFT 2 Choice 2") -> (w4881:u16[])
        n2866 = Array Size(array=w4888) -> (size(s)=w4887:i32)
        n2867 = feedback-in #17(w4881) -> ()
        n2868 = feedback #17(u16[] [100, 100, 100, 100]) -> (w4882:u16[])
        n2869 = feedback-in #18("# Spectra to Ave.") -> ()
        n2870 = feedback #18("# Spectra to Ave.") -> (w4879:dbl)
        n2871 = Not Equal?(x="# Spectra to Ave.", y=w4879) -> (x != y?=w4878:bool)
        n2872 = Not Equal?(x=w4881, y=w4882) -> (x != y?=w4880:bool)
        n2873 = feedback #19(1.0) -> (w4865:dbl)
        n2874 = Compound Arithmetic op=OR("Reset FFT", w4880, w4878) -> (w4863:bool)
        n2875 = Select(t=1.0, s=w4863, f=w4865) -> (s? t:f=w4867:dbl)
        n2876 = Greater?(x=w4867, y="# Spectra to Ave.") -> (0:w4886:bool)
        n2877 = Increment(x=w4867) -> (x+1=w4866:dbl)
        n2878 = feedback-in #19(w4866) -> ()
        n2879 = local read "DMA Update Period (s)"() -> (w4861:dbl)
        n2880 = Multiply(x="# Spectra to Ave.", y=w4861) -> (x*y=→"Ave. Time (s)":dbl)
        n2881 = Build Array(cluster{"f0":dbl, "df":dbl, "magnitude":dbl[]} {"f0"=0.0, "df"=0.0, "magnitude"=[]} ("PSD")) -> (w4870:cluster{"f0":dbl, "df":dbl, "magnitude":dbl[]}[])
        n2882 = Build Array(w4870, w4870, w4870, w4870) -> (w4872:T52)
        n2883 = feedback #20(w4872) -> (w4877:T52)
        n2884 = for {
          N: 4 -> [_]
          tunnel: w4881 -> [w4910] mode=indexing
          tunnel: w4888 -> [w4911]
          tunnel: w4887 -> [w4913]
          tunnel: w4863 -> [w4906]
          tunnel: w4886 -> [w4905]
          tunnel: "# Spectra to Ave." -> [w4904]
          tunnel: [w4903] -> w4876 mode=indexing
          tunnel: w4877 -> [w4908] mode=indexing
          tunnel: [w4907] -> w4864 mode=indexing
          tunnel: w4867 -> [w4902]
          n2885 = Less?(x=w4910, y=w4913) -> (x < y?=w4912:bool)
          n2886 = Index Array(array=w4911, index=w4910) -> (element=w4909:waveform(dbl))
          n2887 = case shown="True" w4912 {
            tunnel: w4909 -> [_ w4930]
            tunnel: w4908 -> [w4915 w4928]
            tunnel: [w4915 w4916] -> w4907
            tunnel: w4906 -> [_ w4927]
            tunnel: w4905 -> [_ w4920]
            tunnel: w4904 -> [_ w4919]
            tunnel: [cluster{"f0":dbl, "df":dbl, "magnitude":dbl[]} {"f0"=0.0, "df"=0.0, "magnitude"=[]} ("PSD") w4921] -> w4903
            tunnel: w4902 -> [_ w4918]
            frame False {
            }
            frame True {
              n2888 = call <vilib>:"Std Deviation and Variance.vi"("X"=w4930) -> ("mean"=w4931:dbl)  [unwired: 1 in, 2 out]
              n2889 = Subtract(x=w4930, y=w4931) -> (x-y=w4929:waveform(dbl))
              n2890 = xnode "Spectral Measurements"("Signals"=w4929) -> ("PSD"=w4923:cluster{"f0":dbl, "df":dbl, "magnitude":dbl[]})  [unwired: 1 in, 1 out]
              n2891 = case shown="False" w4927 {
                tunnel: w4928 -> [w4940 _]
                tunnel: [w4936 w4945] -> w4916
                tunnel: w4923 -> [w4939 w4946]
                tunnel: w4920 -> [w4938 _]
                frame False {
                  n2892 = Build Array (concatenate)(w4940, w4939) -> (w4937:cluster{"f0":dbl, "df":dbl, "magnitude":dbl[]}[])
                  n2893 = case shown="True" w4938 {
                    tunnel: w4937 -> [w4941 w4944]
                    tunnel: [w4941 w4942] -> w4936
                    frame False {
                    }
                    frame True {
                      n2894 = Delete From Array(array=w4944, index=0) -> (array with subset deleted=w4942:cluster{"f0":dbl, "df":dbl, "magnitude":dbl[]}[])  [unwired: 1 in, 1 out]
                    }
                  }
                }
                frame True {
                  n2895 = Build Array(w4946) -> (w4945:cluster{"f0":dbl, "df":dbl, "magnitude":dbl[]}[])
                }
              }
              n2896 = for {
                tunnel: w4916 -> [w4935] mode=indexing
                tunnel: [w4934] -> w4926 mode=indexing
                workers-P: _ -> [_]
                n2897 = Unbundle By Name(w4935) -> ("magnitude"=w4934:dbl[])
              }
              n2898 = Transpose 2D Array(2D array=w4926) -> (transposed array=w4925:dbl[][])
              n2899 = for {
                tunnel: w4925 -> [w4933] mode=indexing
                tunnel: [w4932] -> w4924 mode=indexing
                workers-P: _ -> [_]
                n2900 = Add Array Elements(numeric array=w4933) -> (sum=w4932:dbl)
              }
              n2901 = Select(t=w4919, s=w4920, f=w4918) -> (s? t:f=w4917:dbl)
              n2902 = Divide(x=w4924, y=w4917) -> (x/y=w4922:dbl[])
              n2903 = Bundle By Name(cluster=w4923, "magnitude"=w4922) -> (w4921:cluster{"f0":dbl, "df":dbl, "magnitude":dbl[]})
            }
          }
        }
        n2904 = case shown="True" w4863 {
          tunnel: w4864 -> [w4895 w4901]
          tunnel: [w4895 w4896] -> w4862
          frame False {
          }
          frame True {
            n2905 = Array Subset(array=w4901, index (row)=0 ("index"), length (row)=4 ("length"), index (col)=0 ("index"), length (col)=1 ("length")) -> (w4896:T52)
          }
        }
        n2906 = feedback-in #20(w4862) -> ()
        n2907 = Split 1D Array(array=w4876, index=2) -> (first subarray=→"FFT 1":cluster{"f0":dbl, "df":dbl, "magnitude":dbl[]}[], second subarray=→"FFT 2":cluster{"f0":dbl, "df":dbl, "magnitude":dbl[]}[])
      }
    }
    n2908 = case "For plotting results of scanning MCL" shown="True" w3871 {
      tunnel: w3870 -> [_ w4316]
      tunnel: w3800 -> [_ w4412]
      tunnel: w3879 -> [_ _]
      tunnel: w3772 -> [_ w4386]
      tunnel: w3749 -> [_ w4317]
      tunnel: w3748 -> [_ w4290]
      frame False {
      }
      frame True {
        w4297 = u32 0 items=["Horizontal", "Vertical", "Central", "1st Diagonal", "2nd Diagonal"] ("Type of Symmetry")
        w4325 = u32 0 items=["Horizontal", "Vertical", "Central", "1st Diagonal", "2nd Diagonal"] ("Type of Symmetry")
        w4328 = u32 0 items=["Horizontal", "Vertical", "Central", "1st Diagonal", "2nd Diagonal"] ("Type of Symmetry")
        w4357 = u32 0 items=["Horizontal", "Vertical", "Central", "1st Diagonal", "2nd Diagonal"] ("Type of Symmetry")
        n2909 = Index Array(array=w4386, index=10) -> (element=w4392:waveform(dbl))
        n2910 = Index Array(array=w4386, index=11) -> (element=w4389:waveform(dbl))
        n2911 = local read "Cycles/step (MCL)"() -> (w4342:u64)
        n2912 = Index Array(array=w4386, index="Channel") -> (element=w4388:waveform(dbl))
        n2913 = Unbundle(w4290) -> ("New Image"=w4289:T2, "New Image"=w4288:T2, "New Image"=w4287:T2, "New Image"=w4286:T2)
        n2914 = Unbundle By Name(w4392) -> ("Y"=w4344:dbl[])
        n2915 = Unbundle By Name(w4389) -> ("Y"=w4346:dbl[])
        n2916 = Unbundle By Name(w4388) -> ("Y"=w4351:dbl[])
        n2917 = call "downsample 1D array - double.vi"("Ave N"=w4342, "Array In"=w4344) -> ("Array Out"=w4343:dbl[])  [unwired: 1 out]
        n2918 = call "downsample 1D array - double.vi"("Ave N"=w4342, "Array In"=w4346) -> ("Array Out"=w4345:dbl[])  [unwired: 1 out]
        n2919 = call "downsample 1D array - double.vi"("Ave N"=w4342, "Array In"=w4351) -> ("Array Out"=w4350:dbl[])  [unwired: 1 out]
        n2920 = feedback #21(w4412) -> (w4413:dbl[])
        n2921 = Build Array (concatenate)(w4413, w4412) -> (w4394:dbl[])
        n2922 = feedback #22(w4317) -> (w4319:dbl[])
        n2923 = Build Array (concatenate)(w4319, w4317) -> (w4318:dbl[])
        n2924 = local read "Scan steps (MCL)"() -> (w4299:u64)
        n2925 = Select(t=w4412, s=w4316, f=w4394) -> (s? t:f=w4398:dbl[])
        n2926 = feedback-in #21(w4398) -> ()
        n2927 = Select(t=w4317, s=w4316, f=w4318) -> (s? t:f=w4300:dbl[])
        n2928 = feedback-in #22(w4300) -> ()
        n2929 = local read "Scan lines (y)"() -> (w4285:u64)
        n2930 = local read "N APD Samp/step"() -> (w4301:dbl)
        n2931 = feedback #23(w4343) -> (w4400:dbl[])
        n2932 = Build Array (concatenate)(w4400, w4343) -> (w4391:dbl[])
        n2933 = feedback #24(w4350) -> (w4410:dbl[])
        n2934 = Build Array (concatenate)(w4410, w4350) -> (w4409:dbl[])
        n2935 = feedback #25(w4345) -> (w4402:dbl[])
        n2936 = Build Array (concatenate)(w4402, w4345) -> (w4403:dbl[])
        n2937 = Select(t=w4343, s=w4316, f=w4391) -> (s? t:f=w4347:dbl[])
        n2938 = feedback-in #23(w4347) -> ()
        n2939 = Select(t=w4350, s=w4316, f=w4409) -> (s? t:f=w4349:dbl[])
        n2940 = feedback-in #24(w4349) -> ()
        n2941 = Select(t=w4345, s=w4316, f=w4403) -> (s? t:f=w4348:dbl[])
        n2942 = feedback-in #25(w4348) -> ()
        n2943 = Multiply(x=w4299, y=u64 2) -> (x*y=w4284:u64)
        n2944 = call "integrate 1D array interval - double.vi"("Ave N"=w4301, "Array In"=w4300) -> ("Array Out"=w4312:dbl[])  [unwired: 1 out]
        n2945 = call "integrate 1D array interval - double.vi"("Ave N"=w4301, "Array In"=w4398) -> ("Array Out"=w4397:dbl[])  [unwired: 1 out]
        n2946 = Array Size(array=w4312) -> (size(s)=w4313:i32)
        n2947 = Array Size(array=w4397) -> (size(s)=w4399:i32)
        n2948 = Multiply(x=w4285, y=w4284) -> (x*y=w4315:u64)
        n2949 = Multiply(x=w4285, y=w4284) -> (x*y=w4407:u64)
        n2950 = call-poly <vilib>:"Mean.vi"("X"=w4347) -> ("mean"=w4331:dbl)  [unwired: 1 out]
        n2951 = Subtract(x=w4315, y=w4313) -> (x-y=w4306:u64)
        n2952 = call-poly <vilib>:"Mean.vi"("X"=w4349) -> ("mean"=w4336:dbl)  [unwired: 1 out]
        n2953 = call-poly <vilib>:"Mean.vi"("X"=w4348) -> ("mean"=w4334:dbl)  [unwired: 1 out]
        n2954 = call-poly <vilib>:"Mean.vi"("X"=w4312) -> ("mean"=w4303:dbl)  [unwired: 1 out]
        n2955 = Subtract(x=w4407, y=w4399) -> (x-y=w4341:u64)
        n2956 = call-poly <vilib>:"Mean.vi"("X"=w4397) -> ("mean"=w4338:dbl)  [unwired: 1 out]
        n2957 = Initialize Array(1.0 ("element"), w4306) -> (w4302:dbl[])
        n2958 = Initialize Array(1.0 ("element"), w4341) -> (w4332:dbl[])
        n2959 = Multiply(x=w4302, y=w4303) -> (x*y=w4304:dbl[])
        n2960 = Multiply(x=w4332, y=w4334) -> (x*y=w4335:dbl[])
        n2961 = Multiply(x=w4332, y=w4336) -> (x*y=w4337:dbl[])
        n2962 = Multiply(x=w4332, y=w4331) -> (x*y=w4333:dbl[])
        n2963 = Multiply(x=w4332, y=w4338) -> (x*y=w4339:dbl[])
        n2964 = Build Array (concatenate)(w4347, w4333) -> (w4401:dbl[])
        n2965 = Build Array (concatenate)(w4349, w4337) -> (w4405:dbl[])
        n2966 = Build Array (concatenate)(w4348, w4335) -> (w4404:dbl[])
        n2967 = Build Array (concatenate)(w4312, w4304) -> (w4314:dbl[])
        n2968 = Build Array (concatenate)(w4397, w4339) -> (w4406:dbl[])
        n2969 = Reshape Array(w4401, w4285, w4284) -> (w4367:dbl[][])
        n2970 = Reshape Array(w4314, w4285, w4284) -> (w4310:dbl[][])
        n2971 = Reshape Array(w4405, w4285, w4284) -> (w4359:dbl[][])
        n2972 = Reshape Array(w4404, w4285, w4284) -> (w4374:dbl[][])
        n2973 = Reshape Array(w4406, w4285, w4284) -> (w4384:dbl[][])
        n2974 = Array Subset(array=w4374, index (col)=0 ("index"), length (col)=w4299) -> (w4379:dbl[][])  [unwired: 2 in]
        n2975 = Array Subset(array=w4374, index (col)=w4299) -> (w4377:dbl[][])  [unwired: 3 in]
        n2976 = Array Subset(array=w4359, index (col)=0 ("index"), length (col)=w4299) -> (w4365:dbl[][])  [unwired: 2 in]
        n2977 = Array Subset(array=w4359, index (col)=w4299) -> (w4363:dbl[][])  [unwired: 3 in]
        n2978 = Array Subset(array=w4310, index (col)=0 ("index"), length (col)=w4299) -> (w4309:dbl[][])  [unwired: 2 in]
        n2979 = Array Subset(array=w4310, index (col)=w4299) -> (w4307:dbl[][])  [unwired: 3 in]
        n2980 = Array Subset(array=w4384, index (col)=0 ("index"), length (col)=w4299) -> (w4383:dbl[][])  [unwired: 2 in]
        n2981 = Array Subset(array=w4384, index (col)=w4299) -> (w4381:dbl[][])  [unwired: 3 in]
        n2982 = Array Subset(array=w4367, index (col)=0 ("index"), length (col)=w4299) -> (w4372:dbl[][])  [unwired: 2 in]
        n2983 = Array Subset(array=w4367, index (col)=w4299) -> (w4370:dbl[][])  [unwired: 3 in]
        n2984 = for {
          tunnel: w4379 -> [w4421] mode=indexing
          tunnel: [w4420] -> w4378 mode=indexing
          workers-P: _ -> [_]
          n2985 = Reverse 1D Array(array=w4421) -> (reversed array=w4420:dbl[])
        }
        n2986 = for {
          tunnel: w4365 -> [w4417] mode=indexing
          tunnel: [w4416] -> w4364 mode=indexing
          workers-P: _ -> [_]
          n2987 = Reverse 1D Array(array=w4417) -> (reversed array=w4416:dbl[])
        }
        n2988 = for {
          tunnel: w4309 -> [w4415] mode=indexing
          tunnel: [w4414] -> w4308 mode=indexing
          workers-P: _ -> [_]
          n2989 = Reverse 1D Array(array=w4415) -> (reversed array=w4414:dbl[])
        }
        n2990 = for {
          tunnel: w4383 -> [w4423] mode=indexing
          tunnel: [w4422] -> w4382 mode=indexing
          workers-P: _ -> [_]
          n2991 = Reverse 1D Array(array=w4423) -> (reversed array=w4422:dbl[])
        }
        n2992 = for {
          tunnel: w4372 -> [w4419] mode=indexing
          tunnel: [w4418] -> w4371 mode=indexing
          workers-P: _ -> [_]
          n2993 = Reverse 1D Array(array=w4419) -> (reversed array=w4418:dbl[])
        }
        n2994 = Index Array(array=w4384, index (row)=0) -> (element=→"Waveform Graph":dbl[])  [unwired: 1 in]
        n2995 = Add(x=w4378, y=w4377) -> (x+y=w4376:dbl[][])
        n2996 = Add(x=w4364, y=w4363) -> (x+y=w4362:dbl[][])
        n2997 = Add(x=w4308, y=w4307) -> (x+y=w4292:dbl[][])
        n2998 = Add(x=w4382, y=w4381) -> (x+y=w4356:dbl[][])
        n2999 = Add(x=w4371, y=w4370) -> (x+y=w4369:dbl[][])
        n3000 = Divide(x=w4362, y=2) -> (x/y=w4360:dbl[][])
        n3001 = Divide(x=w4376, y=2) -> (x/y=w4321:dbl[][])
        n3002 = Divide(x=w4369, y=2) -> (x/y=w4323:dbl[][])
        n3003 = To Single Precision Float(number=w4356) -> (single precision float=w4355:sgl[][])
        n3004 = Transpose 2D Array(2D array=w4360) -> (transposed array=→"Data map":dbl[][])
        n3005 = To Single Precision Float(number=w4292) -> (single precision float=w4296:sgl[][])
        n3006 = To Single Precision Float(number=w4321) -> (single precision float=w4327:sgl[][])
        n3007 = To Single Precision Float(number=w4323) -> (single precision float=w4324:sgl[][])
        n3008 = call "IMAQ ArrayToImage"("Image Pixels (Float)"=w4355, "Image"=w4289) -> ("Image Out"=w4358:T2)  [unwired: 8 in, 1 out]
        n3009 = call "IMAQ ArrayToImage"("Image Pixels (Float)"=w4296, "Image"=w4288) -> ("Image Out"=w4298:T2)  [unwired: 8 in, 1 out]
        n3010 = call "IMAQ ArrayToImage"("Image Pixels (Float)"=w4327, "Image"=w4287) -> ("Image Out"=w4329:T2)  [unwired: 8 in, 1 out]
        n3011 = call "IMAQ ArrayToImage"("Image Pixels (Float)"=w4324, "Image"=w4286) -> ("Image Out"=w4326:T2)  [unwired: 8 in, 1 out]
        n3012 = call "IMAQ Symmetry"("Type of Symmetry"=w4357, "Image Src"=w4358) -> ("Image Dst Out"=w4353:T2)  [unwired: 3 in, 1 out]
        n3013 = call "IMAQ Symmetry"("Type of Symmetry"=w4297, "Image Src"=w4298) -> ("Image Dst Out"=w4294:T2)  [unwired: 3 in, 1 out]
        n3014 = call "IMAQ Symmetry"("Type of Symmetry"=w4328, "Image Src"=w4329) -> ("Image Dst Out"=→"Detection Laser X":T2)  [unwired: 3 in, 1 out]
        n3015 = call "IMAQ Symmetry"("Type of Symmetry"=w4325, "Image Src"=w4326) -> ("Image Dst Out"=→"Detection Laser Y":T2)  [unwired: 3 in, 1 out]
        n3016 = call "IMAQ Set Simple Calibration"("Calibration Axis Info"=T42 {"Origin Pixel"={"X"=0.0, "Y"=0.0}, "Angle Relative to Horizontal (deg)"=0.0, "Axis Reference"=0}, "Grid Descriptor"=T43 {"X Step"=0.3, "Y Step"=0.3, "Unit"=enum."Undefined"}, "Image"=w4353) -> ("Calibrated Image"=→"APD 1":T2)  [unwired: 7 in, 1 out]
        n3017 = call "IMAQ Set Simple Calibration"("Calibration Axis Info"=T42 {"Origin Pixel"={"X"=0.0, "Y"=0.0}, "Angle Relative to Horizontal (deg)"=0.0, "Axis Reference"=0}, "Grid Descriptor"=T43 {"X Step"=0.3, "Y Step"=0.3, "Unit"=enum."Undefined"}, "Image"=w4294) -> ("Calibrated Image"=→"APD 2":T2)  [unwired: 7 in, 1 out]
      }
    }
    n3018 = Subtract(x=w3754, y="APD 2 Offset") -> (x-y=w3751:waveform(dbl))
    n3019 = Subtract(x=w3756, y="APD 1 Offset") -> (x-y=w3752:waveform(dbl))
    n3020 = Index Array(array=w3770, index=3) -> (element=w3824:waveform(dbl))
    n3021 = Index Array(array=w3770, index=6) -> (element=w3821:waveform(dbl))
    n3022 = Build Array(w3752, w3751) -> (→"APD Chart":waveform(dbl)[])
    n3023 = Array Size(array=w3592) -> (size(s)=w3860:i32)
    n3024 = call <vilib>:"Std Deviation and Variance.vi"("X"=w3593) -> ("standard deviation"=w3763:dbl)  [unwired: 1 in, 2 out]
    n3025 = Add Array Elements(numeric array=w3593) -> (sum=w3765:u32)
    n3026 = Add Array Elements(numeric array=w3592) -> (sum=w3869:u32)
    n3027 = call <vilib>:"Std Deviation and Variance.vi"("X"=w3592) -> ("standard deviation"=w3815:dbl)  [unwired: 1 in, 2 out]
    n3028 = Divide(x="T1 offset_x (mV)", y=1000.0) -> (x/y=w3825:dbl)
    n3029 = Divide(x=w3763, y=w3762) -> (x/y=w3759:dbl)
    "Rate sigma (Hz) 2" <- w3759
    n3030 = Multiply(x=w3762, y=w3860) -> (x*y=w3764:dbl)
    "Int. Time (s)" <- w3764
    n3031 = Divide(x=w3765, y=w3764) -> (x/y=w3760:dbl)
    "APD 2 Rate (Hz)" <- w3760
    n3032 = Divide(x=w3869, y=w3764) -> (x/y=w3813:dbl)
    "APD 1 Rate (Hz)" <- w3813
    n3033 = Divide(x=w3815, y=w3762) -> (x/y=w3814:dbl)
    "Rate sigma (Hz)" <- w3814